vi "一致性测试确认.vi"(0 "Image In":T11=refnum, 1 "Image Dst":T11, 2 "ROI Descriptor (Find Straight Edge 1)":T4={"Global Rectangle"=[508, 1161, 875, 1411], "Contours"=[{"ID"=enum."External", "Type"=12, "Coordinates"=[508, 1161, 875, 1411, 0]}]} {"Contours"."Type" items=["No Selection", "Point", "Line", "Rectangle", "Oval", "Polygon", "Freehand Region", "Annulus", "Unused2", "Unused3", "Broken Line", "Freehand Line", "Rotated Rectangle"]}, 3 "Options (Find Straight Edge 1)":T9={"Search Direction"=0, "Edge Options"={"Edge Polarity"=0, "Kernel Size"=9, "Width"=25, "Minimum Edge Strength"=47.0, "Interpolation Type"=enum."Bilinear Fixed", "Data Processing Method"=enum."Average"}, "Show Search Area"=TRUE, "Show Search Lines"=FALSE, "Show Edges Found"=FALSE, "Show Result"=TRUE, "Search Area Color"=6618880, "Search Lines Color"=16860, "Edge Locations Color"=6618880, "Result Color"=16711680, "Overlay Group Name"=""} {"Search Direction" items=["Left to Right", "Right to Left", "Top to Bottom", "Bottom to Top"]; "Edge Options"."Edge Polarity" items=["All Edges", "Rising Edges", "Falling Edges"]; "Edge Options"."Minimum Edge Strength" format="%.2f"; "Edge Options"."Width" step=2; "Edge Options"."Kernel Size" step=2}, 4 "Fit Options (Find Straight Edge 1)":T5={"Number of Lines"=1, "Type"=enum."First Edge Rake", "Min. Score"=10.0, "Max. Score"=1000.0, "Orientation"=0.0, "Angle Range"=45.0, "Angle Tolerance"=1.0, "Step Size"=12, "Min. SNR (db)"=0.0, "Min. Points (%)"=25.0, "Hough Iterations"=5} {"Min. Points (%)" min=0.0 max=100.0; "Min. SNR (db)" min=0.0; "Max. Score" min=0.0 max=1024.0; "Min. Score" min=0.0 max=1024.0 step=1.0}, 5 "ROI Descriptor (Edge Detector 1)":T4={"Global Rectangle"=[710, 1241, 2012, 1251], "Contours"=[{"ID"=enum."External", "Type"=2, "Coordinates"=[710, 1250, 2011, 1241]}]} {"Contours"."Type" items=["No Selection", "Point", "Line", "Rectangle", "Oval", "Polygon", "Freehand Region", "Annulus", "Unused2", "Unused3", "Broken Line", "Freehand Line", "Rotated Rectangle"]}, 6 "Process (Edge Detector 1)":T3(ring)=enum."Get All Edges", 7 "error in":errorcluster, 8 "Edge Options (Edge Detector 1)":T2={"Edge Polarity"=0, "Kernel Size"=9, "Width"=25, "Minimum Edge Strength"=47.0, "Interpolation Type"=enum."Bilinear Fixed", "Data Processing Method"=enum."Average"} {"Edge Polarity" items=["All Edges", "Rising Edges", "Falling Edges"]}, 9 "Algorithm (Pattern Matching 1)":i32(ring)=2 items=["All", "Low Discrepancy Sampling", "Grayscale Value Pyramid", "Gradients Pyramid"], 10 "Parameters (Pattern Matching 1)":T10={"Number of Matches Requested"=1, "Minimum Match Score"=699.0, "Angle Ranges"=[{"Start Angle"=-20.0, "End Angle"=20.0}]}, 11 "Template File Path (Pattern Matching 1)":path=path "D:/Inspect System/Source Code/Template Program/一致性模板.png", 12 "ROI Descriptor (Find Straight Edge 2)":T4={"Global Rectangle"=[1843, 1112, 2152, 1339], "Contours"=[{"ID"=enum."External", "Type"=12, "Coordinates"=[1844, 1113, 2151, 1338, -262]}]} {"Contours"."Type" items=["No Selection", "Point", "Line", "Rectangle", "Oval", "Polygon", "Freehand Region", "Annulus", "Unused2", "Unused3", "Broken Line", "Freehand Line", "Rotated Rectangle"]}, 13 "Options (Find Straight Edge 2)":T9={"Search Direction"=1, "Edge Options"={"Edge Polarity"=1, "Kernel Size"=7, "Width"=1, "Minimum Edge Strength"=51.0, "Interpolation Type"=enum."Bilinear Fixed", "Data Processing Method"=enum."Average"}, "Show Search Area"=TRUE, "Show Search Lines"=FALSE, "Show Edges Found"=FALSE, "Show Result"=TRUE, "Search Area Color"=65280, "Search Lines Color"=255, "Edge Locations Color"=16776960, "Result Color"=16711680, "Overlay Group Name"=""} {"Search Direction" items=["Left to Right", "Right to Left", "Top to Bottom", "Bottom to Top"]; "Edge Options"."Edge Polarity" items=["All Edges", "Rising Edges", "Falling Edges"]; "Edge Options"."Minimum Edge Strength" format="%.2f"; "Edge Options"."Width" step=2; "Edge Options"."Kernel Size" step=2}, 14 "Fit Options (Find Straight Edge 2)":T5={"Number of Lines"=1, "Type"=enum."First Edge Rake", "Min. Score"=10.0, "Max. Score"=1000.0, "Orientation"=0.0, "Angle Range"=45.0, "Angle Tolerance"=1.0, "Step Size"=7, "Min. SNR (db)"=0.0, "Min. Points (%)"=25.0, "Hough Iterations"=5} {"Min. Points (%)" min=0.0 max=100.0; "Min. SNR (db)" min=0.0; "Max. Score" min=0.0 max=1024.0; "Min. Score" min=0.0 max=1024.0 step=1.0}) -> (20 "Image Out":T11, 21 "Edge Information (Edge Detector 1)":T12[](array[typedef])=[{"Location (Pixel)"={"X"=1992.7675, "Y"=1249.6696}, "Location (Real-World)"={"X"=1992.7675, "Y"=1249.6696}, "Distance (Pixel)"=1243.7788960188627, "Distance (Real-World)"=1243.7788960188627, "Strength"=48.61714285714286, "Noise"=33.48, "Rising?"=FALSE}, {"Location (Pixel)"={"X"=2093.2168, "Y"=1249.239}, "Location (Real-World)"={"X"=2093.2168, "Y"=1249.239}, "Distance (Pixel)"=1344.2292914241552, "Distance (Real-World)"=1344.2292914241552, "Strength"=135.82857142857142, "Noise"=25.725714285714286, "Rising?"=FALSE}] {"Distance (Real-World)" format="%.2f"; "Location (Real-World)"."Y" format="%.2g"; "Location (Real-World)"."X" format="%.2f"; "Noise" format="%.2f"; "Location (Pixel)"."Y" format="%.2g"; "Location (Pixel)"."X" format="%.2f"; "Strength" format="%.2f"; "Distance (Pixel)" format="%.2f"}, 22 "Straight Edge (Find Straight Edge 1)":T13={"Point1 (Pixels)"={"X"=694.03955, "Y"=1165.1874}, "Point2 (Pixels)"={"X"=693.5, "Y"=1405.0}, "Point1 (Real-World)"={"X"=694.03955, "Y"=1165.1874}, "Point2 (Real-World)"={"X"=693.5, "Y"=1405.0}, "Angle (Pixel)"=-0.12890037757524908, "Angle (Real-World)"=-0.12890037757524908, "Score"=261.62465413411456, "Straightness"=0.11302218027687676, "Average SNR (db)"=31.042020668112016, "Calibration Valid"=TRUE} {"Point2 (Real-World)"."Y" format="%.2f"; "Point2 (Real-World)"."X" format="%.2f"; "Point1 (Real-World)"."Y" format="%.2f"; "Point1 (Real-World)"."X" format="%.2f"; "Point2 (Pixels)"."Y" format="%.2f"; "Point2 (Pixels)"."X" format="%.2f"; "Point1 (Pixels)"."Y" format="%.2f"; "Point1 (Pixels)"."X" format="%.2f"}, 23 "Matches (Pattern Matching 1)":T14(array[cluster])=[{"Position"={"x"=1379.1647, "y"=1245.8256}, "Angle"=0.08344074, "Scale"=1.0, "Score"=860.556, "Bounding Box"=[{"x"=653.5562, "y"=1171.8822}, {"x"=2104.5547, "y"=1169.7692}, {"x"=2104.773, "y"=1319.7689}, {"x"=653.7747, "y"=1321.882}, {"x"=653.5562, "y"=1171.8822}]}] {"Bounding Box"."y" format="%.2f"; "Bounding Box"."x" format="%.2f"; "Position"."y" format="%.2f"; "Position"."x" format="%.2f"; "Score" format="%.2f"; "Scale" format="%.2f"; "Angle" format="%.2f"}, 24 "Straight Edge (Find Straight Edge 2)":T13={"Point1 (Pixels)"={"X"=2089.7798, "Y"=1115.0}, "Point2 (Pixels)"={"X"=2095.6719, "Y"=1339.0}, "Point1 (Real-World)"={"X"=2089.7798, "Y"=1115.0}, "Point2 (Real-World)"={"X"=2095.6719, "Y"=1339.0}, "Angle (Pixel)"=1.5067815290214939, "Angle (Real-World)"=1.5067815290214939, "Score"=227.45098039215685, "Straightness"=2.5179862328858427, "Average SNR (db)"=23.738052089260176, "Calibration Valid"=TRUE} {"Point2 (Real-World)"."Y" format="%.2f"; "Point2 (Real-World)"."X" format="%.2f"; "Point1 (Real-World)"."Y" format="%.2f"; "Point1 (Real-World)"."X" format="%.2f"; "Point2 (Pixels)"."Y" format="%.2f"; "Point2 (Pixels)"."X" format="%.2f"; "Point1 (Pixels)"."Y" format="%.2f"; "Point1 (Pixels)"."X" format="%.2f"}, 25 "输出簇":T1={"Start X"=694, "Start Y"=1250, "End X"=2093, "End Y"=1241} {"Start X" scale=0.0..1024.0; "End X" scale=0.0..1024.0}, 27 "error out":errorcluster)   [LabVIEW 2017]
doc: "Creates, edits, and runs vision algorithms using NI Vision Assistant.\n\nWhen you place this Express VI on the block diagram, NI Vision Assistant launches. Create an algorithm using the Vision Assistant processing functions. After you create an algorithm, you can select the controls and indicators that you want to be able to programmatically set in LabVIEW. Double-click the Vision Assistant Express VI to edit the algorithm."
uses:
  <vilib>/vision/Image Controls.llb/IMAQ Image.ctl
  <vilib>/vision/Measure.llb/Edge New.ctl
  <vilib>/vision/Measure.llb/Edge Options.ctl
  <vilib>/vision/Measure.llb/Edge Polarity.ctl
  <vilib>/vision/Measure.llb/Straight Edge Options.ctl
  <vilib>/vision/Measure.llb/Straight Edge Process.ctl
  <vilib>/vision/NI_Vision_Development_Module.lvlib
panel:
  out "end X":sgl=2092.7258
  out "start X":sgl=693.7698
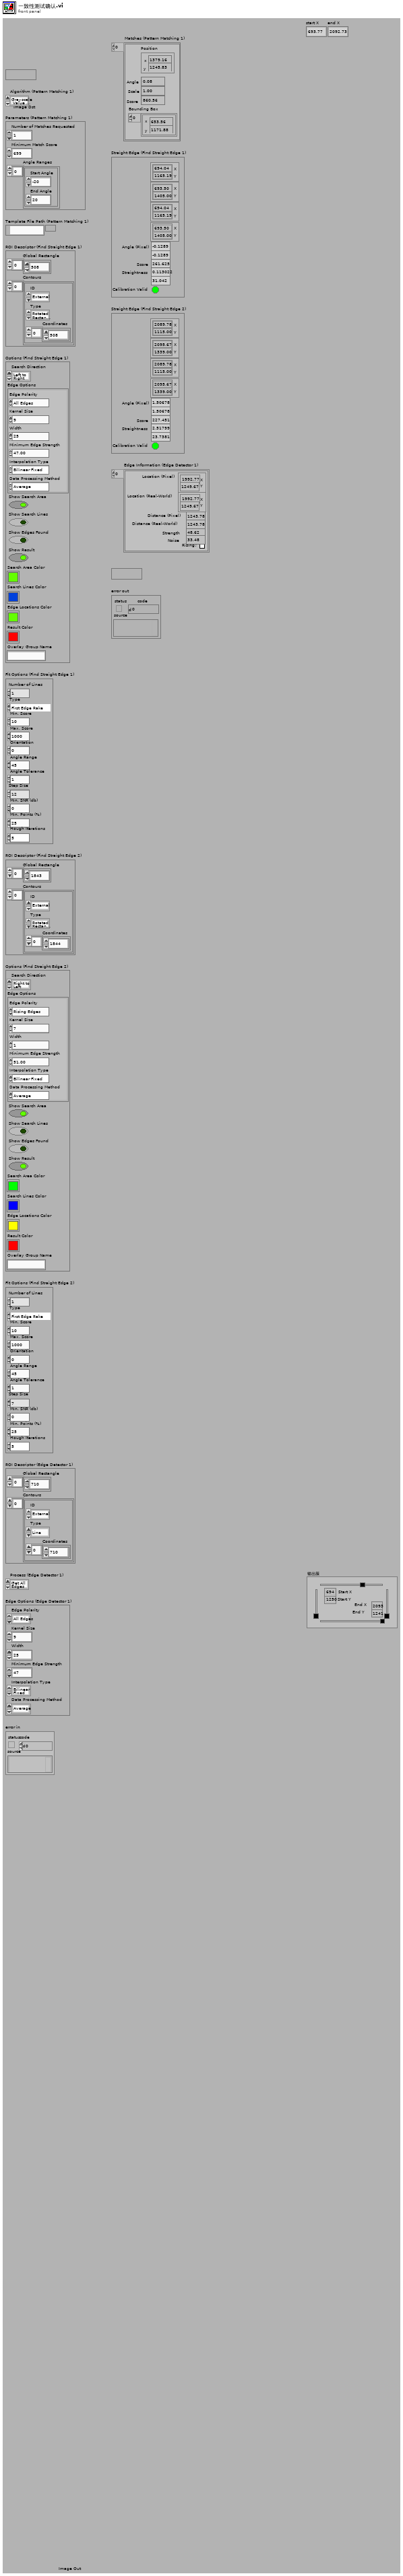
[diagram p1: front panel]
types:
  T1 = typedef "IMAQ Line" = cluster{"Start X":i32, "Start Y":i32, "End X":i32, "End Y":i32}
  T2 = cluster{"Edge Polarity":u32, "Kernel Size":u32, "Width":u32, "Minimum Edge Strength":sgl, "Interpolation Type":enum32{"Zero Order", "Bilinear", "Quadratic", "Cubic", "Bilinear Fixed"}, "Data Processing Method":enum32{"Average", "Median"}}
  T3 = enum16{"Get First Edge", "Get First + Last Edge", "Get All Edges", "Get Best Edge"}
  T4 = cluster{"Global Rectangle":i32[], "Contours":cluster{"ID":enum32{"External", "Internal"}, "Type":u32, "Coordinates":i32[]}[]}
  T5 = typedef "Straight Edge Options.ctl" = cluster{"Number of Lines":i32, "Type":T6, "Min. Score":dbl, "Max. Score":dbl, "Orientation":dbl, "Angle Range":dbl, "Angle Tolerance":dbl, "Step Size":u32, "Min. SNR (db)":dbl, "Min. Points (%)":dbl, "Hough Iterations":i32}
  T6 = typedef "Straight Edge Process.ctl" = enum32{"First Edge Rake", "Best Edge Rake", "Hough Edge Rake", "First Edge Projection", "Best Edge Projection"}
  T7 = typedef "Edge Options.ctl" = cluster{"Edge Polarity":T8, "Kernel Size":u32, "Width":u32, "Minimum Edge Strength":sgl, "Interpolation Type":enum32{"Zero Order", "Bilinear", "Quadratic", "Cubic", "Bilinear Fixed"}, "Data Processing Method":enum32{"Average", "Median"}}
  T8 = typedef "Edge Polarity.ctl" = u32
  T9 = cluster{"Search Direction":u32, "Edge Options":T7, "Show Search Area":bool, "Show Search Lines":bool, "Show Edges Found":bool, "Show Result":bool, "Search Area Color":u32, "Search Lines Color":u32, "Edge Locations Color":u32, "Result Color":u32, "Overlay Group Name":string}
  T10 = cluster{"Number of Matches Requested":i32, "Minimum Match Score":sgl, "Angle Ranges":cluster{"Start Angle":sgl, "End Angle":sgl}[]}
  T11 = typedef "IMAQ Image.ctl" = refnum<image>
  T12 = typedef "Edge New.ctl" = cluster{"Location (Pixel)":cluster{"X":sgl, "Y":sgl}, "Location (Real-World)":cluster{"X":sgl, "Y":sgl}, "Distance (Pixel)":dbl, "Distance (Real-World)":dbl, "Strength":dbl, "Noise":dbl, "Rising?":bool}
  T13 = cluster{"Point1 (Pixels)":cluster{"X":sgl, "Y":sgl}, "Point2 (Pixels)":cluster{"X":sgl, "Y":sgl}, "Point1 (Real-World)":cluster{"X":sgl, "Y":sgl}, "Point2 (Real-World)":cluster{"X":sgl, "Y":sgl}, "Angle (Pixel)":dbl, "Angle (Real-World)":dbl, "Score":dbl, "Straightness":dbl, "Average SNR (db)":dbl, "Calibration Valid":bool}
  T14 = cluster{"Position":cluster{"x":sgl, "y":sgl}, "Angle":sgl, "Scale":sgl, "Score":sgl, "Bounding Box":cluster{"x":sgl, "y":sgl}[]}[]
  T15 = cluster{"Origin":cluster{"X":sgl, "Y":sgl}, "Angle (deg)":sgl, "Axis Reference":u32}
  T16 = enum16{"Reset", "Update Coordinate System", "Get Coordinate System"}
  T17 = enum16{"Horizontal Motion", "Vertical Motion", "Horizontal and Vertical Motion", "Horizontal, Vertical and Angular Motion"}
  T18 = typedef "Image Type" = u32
  T19 = typedef "IMAQ Coordinate System" = cluster{"Reference System":cluster{"Origin":cluster{"X":sgl, "Y":sgl}, "Angle (deg)":sgl, "Axis Reference":u32}, "Measurement System":cluster{"Origin":cluster{"X":sgl, "Y":sgl}, "Angle (deg)":sgl, "Axis Reference":u32}}
  T20 = typedef "ROI Descriptor" = cluster{"Global Rectangle":i32[], "Contours":cluster{"ID":enum32{"External", "Internal"}, "Type":u32, "Coordinates":i32[]}[]}
  T21 = cluster{"Point1 (Pixels)":cluster{"X":sgl, "Y":sgl}, "Point2 (Pixels)":cluster{"X":sgl, "Y":sgl}, "Point1 (Real-World)":cluster{"X":sgl, "Y":sgl}, "Point2 (Real-World)":cluster{"X":sgl, "Y":sgl}, "Angle (Pixel)":dbl, "Angle (Real-World)":dbl, "Score":dbl, "Straightness":dbl, "Average SNR (db)":dbl, "Calibration Valid":bool}[]
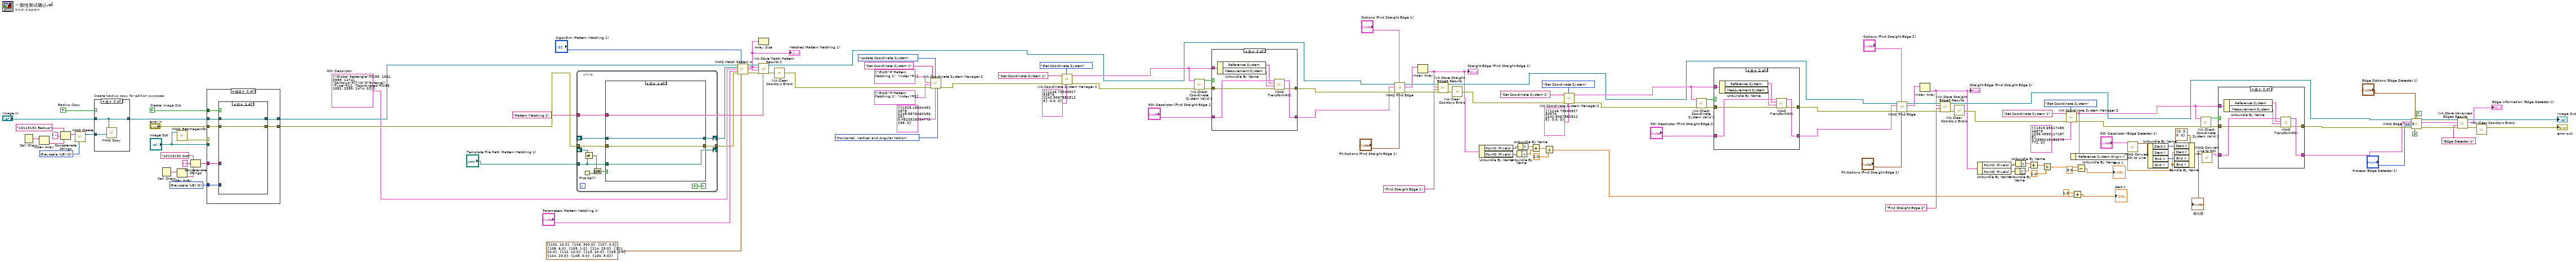
[diagram p0: block diagram]
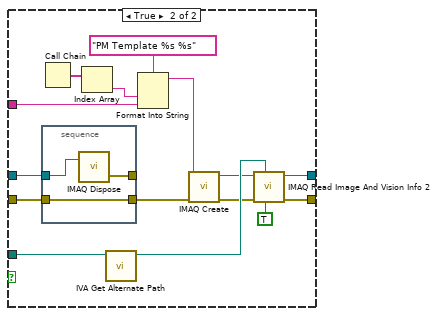
[diagram p5: hidden frame]
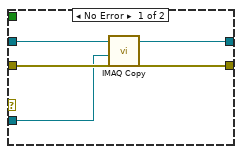
[diagram p6: hidden frame]
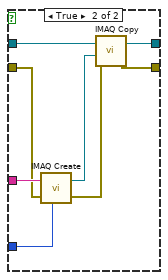
[diagram p7: hidden frame]
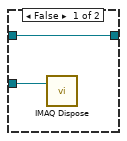
[diagram p8: hidden frame]
diagram:
  w103 = "Pattern Matching 1" ("Step Name")
  w105 = T4 {"Global Rectangle"=[295, 1061, 2595, 1474], "Contours"=[{"ID"=enum."External", "Type"=12, "Coordinates"=[295, 1061, 2595, 1474, 0]}]}  # ROI Descriptor
  w111 = T18 0 items=["Grayscale (U8)", "Grayscale (I16)", "Grayscale (SGL)", "Complex (CSG)", "RGB (U32)", "HSL (U32)", "RGB (U64)", "Grayscale (U16)"] ("Image Dst Type")
  w112 = T18 0 items=["Grayscale (U8)", "Grayscale (I16)", "Grayscale (SGL)", "Complex (CSG)", "RGB (U32)", "HSL (U32)", "RGB (U64)", "Grayscale (U16)"] ("Image Type")
  w131 = TRUE  # Backup Copy
  w124 = FALSE  # Create Image Dst
  n1 = Call Chain() -> (call chain=w118:string[])
  n2 = Index Array(array=w118) -> (element=w117:string)  [unwired: 1 in]
  n3 = Concatenate Strings("10113132 Backup" ("Backup Image Name"), " ", w117) -> (w114:string)
  n4 = call "IMAQ Create"("Image Name"=w114, "Image Type"=w112) -> ("New Image"=w113:T11)  [unwired: 2 in, 2 out]
  n5 = case "Create backup copy for edition purposes" shown="真" w131 {
    tunnel: [w133 w135] -> w127
    tunnel: "Image In" -> [w133 w135]
    tunnel: w113 -> [w132 w134]
    frame False {
      n6 = call "IMAQ Dispose"("Image"=w132) -> ()  [unwired: 2 in, 4 out]
    }
    frame True {
      n7 = call "IMAQ Copy"("Image Dst"=w134, "Image Src"=w135) -> ()  [unwired: 1 in, 5 out]
    }
  }
  n8 = Call Chain() -> (call chain=w123:string[])
  n9 = call "IMAQ GetImageInfo"("Image"="Image Dst") -> ("error out"=w129:errorcluster)  [unwired: 1 in, 9 out]
  n10 = Index Array(array=w123) -> (element=w121:string)  [unwired: 1 in]
  n11 = Concatenate Strings("10113132 Dst" ("Image Dst Name"), " ", w121) -> (w119:string)
  n12 = case "条件结构" shown="错误" w129 {
    tunnel: [w140 w144] -> w109
    tunnel: [w139 w143] -> w125
    tunnel: w127 -> [w138 w145]
    tunnel: "error in" -> [w137 w141]
    tunnel: "Image Dst" -> [w136 _]
    tunnel: w119 -> [_ w147]
    tunnel: w111 -> [_ w146]
    tunnel: w124 -> [_ w142]
    frame No Error {
      n13 = call "IMAQ Copy"("error in (no error)"=w137, "Image Dst"=w136, "Image Src"=w138) -> ("error out"=w139:errorcluster, "Image Dst Out"=w140:T11)  [unwired: 3 out]
    }
    frame Error {
      n14 = case "条件结构" shown="假" w142 {
        tunnel: w147 -> [_ w157]
        tunnel: w146 -> [_ w156]
        tunnel: w145 -> [w149 w154]
        tunnel: [w149 w153] -> w144
        tunnel: [w148 w152] -> w143
        tunnel: w141 -> [w148 w150]
        frame False {
        }
        frame True {
          n15 = call "IMAQ Create"("Image Name"=w157, "Image Type"=w156, "error in (no error)"=w150) -> ("New Image"=w155:T11, "error out"=w151:errorcluster)  [unwired: 1 in, 1 out]
          n16 = call "IMAQ Copy"("error in (no error)"=w151, "Image Dst"=w155, "Image Src"=w154) -> ("error out"=w152:errorcluster, "Image Dst Out"=w153:T11)  [unwired: 3 out]
        }
      }
    }
  }
  n17 = while {
    shift-right: [w168] -> w100
    shift-left: _ -> [w167]
    tunnel: [w165] -> w99
    tunnel: w125 -> [w164]
    tunnel: "Template File Path (Pattern Matching 1)" -> [w161]
    tunnel: w103 -> [w163]
    shift-right: [w161] -> _
    shift-left: _ -> [w162]
    stop <- FALSE continue-if-true
    n18 = First Call?() -> (First Call?: T/F=w160:bool)
    n19 = Not Equal?(x=w162, y=w161) -> (x != y?=w159:bool)
    n20 = Or(x=w159, y=w160) -> (x .or. y?=w158:bool)
    n21 = case "条件结构" shown="假" w158 {
      tunnel: [w170 w175] -> w168
      tunnel: w167 -> [w170 w179]
      tunnel: [w169 w176] -> w165
      tunnel: w164 -> [w169 w178]
      tunnel: w161 -> [_ w180]
      tunnel: w163 -> [_ w181]
      frame False {
      }
      frame True {
        n22 = stacked-sequence "层叠式顺序结构" {
          tunnel: w179 -> [w188]
          tunnel: w178 -> [w187]
          tunnel: [w187] -> w172
          tunnel: [w186] -> _
          frame #0 {
            n23 = call "IMAQ Dispose"("Image"=w188) -> ("error out"=w186:errorcluster)  [unwired: 2 in, 3 out]
          }
        }
        n24 = Call Chain() -> (call chain=w183:string[])
        n25 = Index Array(array=w183) -> (element=w182:string)  [unwired: 1 in]
        n26 = call <vilib>:"IVA Get Alternate Path.vi"("Path In"=w180) -> ("Path Out"=w177:path)  [unwired: 10 out]
        n27 = Format Into String(format string="PM Template %s %s" ("Image Name"), w182, w181) -> (resulting string=w185:string)  [unwired: 2 in, 1 out]
        n28 = call "IMAQ Create"("Image Name"=w185, "error in (no error)"=w172) -> ("New Image"=w174:T11, "error out"=w173:errorcluster)  [unwired: 2 in, 1 out]
        n29 = call "IMAQ Read Image And Vision Info 2"("Use File Path Image Type"=TRUE, "File Path"=w177, "error in (no error)"=w173, "Image"=w174) -> ("error out"=w176:errorcluster, "Image Out"=w175:T11)  [unwired: 5 in, 1 out]
      }
    }
  }
  n30 = call "IMAQ Match Pattern 4"("Image"=w109, "Algorithm"="Algorithm (Pattern Matching 1)", "Template Image"=w100, "ROI Descriptor"=w105, "Parameters"="Parameters (Pattern Matching 1)", "error in (no error)"=w99, "Advanced Options"=cluster{"Item":u16, "Value":dbl}[] [{"Item"=102, "Value"=10.0}, {"Item"=106, "Value"=300.0}, {"Item"=107, "Value"=0.0}, {"Item"=108, "Value"=6.0}, {"Item"=109, "Value"=1.0}, {"Item"=114, "Value"=25.0}, {"Item"=111, "Value"=20.0}, {"Item"=112, "Value"=10.0}, {"Item"=113, "Value"=20.0}, {"Item"=103, "Value"=1.0}, {"Item"=104, "Value"=20.0}, {"Item"=105, "Value"=0.0}, {"Item"=100, "Value"=5.0}]) -> ("Image (duplicate)"=w107:T11, "Matches (pixel)"=w102:T14, "Matches (real-world)"=w101:T14, "error out"=w108:errorcluster)  [unwired: 4 in, 1 out]
  "Matches (Pattern Matching 1)" <- w102
  n31 = Array Size(array=w102) -> ()  [unwired: 1 out]
  n32 = call <vilib>:"IVA Store Match Pattern Results 2.vi"("Step Name"=w103, "error in (no error)"=w108, "Matches (real-world)"=w101, "Matches (pixel)"=w102, "Image in"=w107) -> ("error out"=w98:errorcluster, "Image dup"=w79:T11)  [unwired: 1 in, 4 out]
  n33 = call <vilib>:"IVA Clear Coordsys Errors.vi"("error in (no error)"=w98) -> ("error out"=w97:errorcluster)  [unwired: 10 in]
  n34 = call <vilib>:"IVA Coordinate System Manager 2.vi"("Mode"=T17."Horizontal, Vertical and Angular Motion", "Reference System"=T15 {"Origin"={"X"=1329.196, "Y"=1248.8577}, "Angle (deg)"=0.45203266, "Axis Reference"=0}, "Function"=T16."Update Coordinate System", "error in (no error)"=w97, "Angle ID"=cluster{"GUID":string, "Index":i32} {"GUID"="Pattern Matching 1", "Index"=3}, "Origin ID"=cluster{"GUID":string, "Index":i32} {"GUID"="Pattern Matching 1", "Index"=1}, "Coordinate System Name"="Set Coordinate System 1") -> ("error out"=w89:errorcluster)  [unwired: 4 out]
  n35 = call <vilib>:"IVA Coordinate System Manager 2.vi"("Reference System"=T15 {"Origin"={"X"=1246.7904, "Y"=1242.9067}, "Angle (deg)"=0.0, "Axis Reference"=0}, "Function"=T16."Get Coordinate System", "error in (no error)"=w89, "Coordinate System Name"="Set Coordinate System 1") -> ("error out"=w86:errorcluster, "Coordinate System Out"=w82:T19)  [unwired: 3 in, 3 out]
  n36 = call <vilib>:"IVA Check Coordinate System Valid 2.vi"("error in (no error)"=w86, "Coordinate System"=w82) -> ("error out"=w80:errorcluster, "Valid?"=w81:bool)  [unwired: 8 out]
  n37 = case "条件结构" shown="真" w81 {
    tunnel: "ROI Descriptor (Find Straight Edge 1)" -> [w190 w197]
    tunnel: [w190 w194] -> w78
    tunnel: [w189 w193] -> w83
    tunnel: w82 -> [_ w192]
    tunnel: w80 -> [w189 w191]
    frame False {
    }
    frame True {
      n38 = Unbundle By Name(w192) -> ("Reference System"=w196:T15, "Measurement System"=w195:T15)
      n39 = call "IMAQ TransformROI"("error in (no error)"=w191, "New Reference"=w195, "Base Reference"=w196, "ROI Descriptor"=w197) -> ("error out"=w193:errorcluster, "ROI Descriptor out"=w194:T20)  [unwired: 6 out]
    }
  }
  n40 = call "IMAQ Find Edge"("Line Fit Options"="Fit Options (Find Straight Edge 1)", "Options"="Options (Find Straight Edge 1)", "error in (no error)"=w83, "ROI Descriptor"=w78, "Image"=w79) -> ("error out"=w73:errorcluster, "Straight Edges"=w72:T21, "Image Out"=w74:T11)  [unwired: 1 in, 3 out]
  n41 = Index Array(array=w72) -> (element=w24:T13)  [unwired: 1 in]
  "Straight Edge (Find Straight Edge 1)" <- w24
  n42 = call <vilib>:"IVA Store Straight Edge3 Results.vi"("error in (no error)"=w73, "Step Name"="Find Straight Edge 1", "Straight Edge"=w24, "Image in"=w74) -> ("error out"=w71:errorcluster, "Image dup"=w60:T11)  [unwired: 1 in, 5 out]
  n43 = call <vilib>:"IVA Clear Coordsys Errors.vi"("error in (no error)"=w71) -> ("error out"=w70:errorcluster)  [unwired: 10 in]
  n44 = Unbundle By Name(w24) -> ("Point1 (Pixels)"=w29:cluster{"X":sgl, "Y":sgl}, "Point2 (Pixels)"=w28:cluster{"X":sgl, "Y":sgl})
  n45 = Unbundle By Name(w28) -> ("X"=w26:sgl)
  n46 = Unbundle By Name(w29) -> ("X"=w27:sgl)
  n47 = Add(x=w27, y=w26) -> (x+y=w25:sgl)
  n48 = Divide(x=w25, y=sgl 2.0) -> (x/y=w10:sgl)
  n49 = call <vilib>:"IVA Coordinate System Manager 2.vi"("Reference System"=T15 {"Origin"={"X"=1246.7904, "Y"=1242.9067}, "Angle (deg)"=0.0, "Axis Reference"=0}, "Function"=T16."Get Coordinate System", "error in (no error)"=w70, "Coordinate System Name"="Set Coordinate System 1") -> ("error out"=w67:errorcluster, "Coordinate System Out"=w63:T19)  [unwired: 3 in, 3 out]
  n50 = call <vilib>:"IVA Check Coordinate System Valid 2.vi"("error in (no error)"=w67, "Coordinate System"=w63) -> ("error out"=w61:errorcluster, "Valid?"=w62:bool)  [unwired: 8 out]
  n51 = case "条件结构" shown="真" w62 {
    tunnel: "ROI Descriptor (Find Straight Edge 2)" -> [w199 w206]
    tunnel: [w199 w203] -> w59
    tunnel: [w198 w202] -> w64
    tunnel: w63 -> [_ w201]
    tunnel: w61 -> [w198 w200]
    frame False {
    }
    frame True {
      n52 = Unbundle By Name(w201) -> ("Reference System"=w205:T15, "Measurement System"=w204:T15)
      n53 = call "IMAQ TransformROI"("error in (no error)"=w200, "New Reference"=w204, "Base Reference"=w205, "ROI Descriptor"=w206) -> ("error out"=w202:errorcluster, "ROI Descriptor out"=w203:T20)  [unwired: 6 out]
    }
  }
  n54 = call "IMAQ Find Edge"("Line Fit Options"="Fit Options (Find Straight Edge 2)", "Options"="Options (Find Straight Edge 2)", "error in (no error)"=w64, "ROI Descriptor"=w59, "Image"=w60) -> ("error out"=w54:errorcluster, "Straight Edges"=w53:T21, "Image Out"=w55:T11)  [unwired: 1 in, 3 out]
  n55 = Index Array(array=w53) -> (element=w16:T13)  [unwired: 1 in]
  "Straight Edge (Find Straight Edge 2)" <- w16
  n56 = call <vilib>:"IVA Store Straight Edge3 Results.vi"("error in (no error)"=w54, "Step Name"="Find Straight Edge 2", "Straight Edge"=w16, "Image in"=w55) -> ("error out"=w52:errorcluster, "Image dup"=w43:T11)  [unwired: 1 in, 5 out]
  n57 = call <vilib>:"IVA Clear Coordsys Errors.vi"("error in (no error)"=w52) -> ("error out"=w51:errorcluster)  [unwired: 10 in]
  n58 = Unbundle By Name(w16) -> ("Point1 (Pixels)"=w17:cluster{"X":sgl, "Y":sgl}, "Point2 (Pixels)"=w18:cluster{"X":sgl, "Y":sgl})
  n59 = Unbundle By Name(w18) -> ("X"=w20:sgl)
  n60 = Unbundle By Name(w17) -> ("X"=w19:sgl)
  n61 = Add(x=w19, y=w20) -> (x+y=w21:sgl)
  n62 = Divide(x=w21, y=sgl 2.0) -> (x/y=w11:sgl)
  n63 = call <vilib>:"IVA Coordinate System Manager 2.vi"("Reference System"=T15 {"Origin"={"X"=1323.6542, "Y"=1239.4995}, "Angle (deg)"=0.23892452, "Axis Reference"=0}, "Function"=T16."Get Coordinate System", "error in (no error)"=w51, "Coordinate System Name"="Set Coordinate System 1") -> ("error out"=w48:errorcluster, "Coordinate System Out"=w4:T19)  [unwired: 3 in, 3 out]
  n64 = Unbundle By Name(w4) -> ("Reference System.Origin.Y"=w3:sgl)
  n65 = Add(x=sgl 1.0, y=w10) -> (x+y=→"start X":sgl)
  n66 = Subtract(x=w11, y=sgl 5.0) -> (x-y=→"end X":sgl)
  n67 = call "IMAQ Convert ROI to Line"("ROI Descriptor"="ROI Descriptor (Edge Detector 1)") -> ("Line"=w14:T1)  [unwired: 8 in, 1 out]
  n68 = Unbundle By Name(w14) -> ("Start X"=w2:i32, "End X"=w1:i32)  [unwired: 2 out]
  n69 = Bundle By Name(cluster=T1 {"Start X"=0, "Start Y"=0, "End X"=0, "End Y"=0} ("Line"), "Start X"=w2, "Start Y"=w3, "End X"=w1, "End Y"=w3) -> (w13:T1)
  "输出簇" <- w13
  n70 = call <vilib>:"IVA Check Coordinate System Valid 2.vi"("error in (no error)"=w48, "Coordinate System"=w4) -> ("error out"=w44:errorcluster, "Valid?"=w45:bool)  [unwired: 8 out]
  n71 = call "IMAQ Convert Line to ROI"("Line"=w13) -> ("ROI Descriptor"=w9:T20)  [unwired: 8 in, 1 out]
  n72 = case "条件结构" shown="真" w45 {
    tunnel: w9 -> [w208 w215]
    tunnel: [w208 w212] -> w35
    tunnel: [w207 w211] -> w46
    tunnel: w4 -> [_ w210]
    tunnel: w44 -> [w207 w209]
    frame False {
    }
    frame True {
      n73 = Unbundle By Name(w210) -> ("Reference System"=w214:T15, "Measurement System"=w213:T15)
      n74 = call "IMAQ TransformROI"("error in (no error)"=w209, "New Reference"=w213, "Base Reference"=w214, "ROI Descriptor"=w215) -> ("error out"=w211:errorcluster, "ROI Descriptor out"=w212:T20)  [unwired: 6 out]
    }
  }
  n75 = call "IMAQ Edge Tool 3"("Image"=w43, "Edge Options"="Edge Options (Edge Detector 1)", "Optimized Mode"=TRUE, "ROI Descriptor"=w35, "Process"="Process (Edge Detector 1)", "error in (no error)"=w46, "Reverse Direction"=FALSE) -> ("Image (duplicate)"=w39:T11, "Edge Information"=w38:T12[], "error out"=w40:errorcluster)  [unwired: 6 out]
  n76 = call <vilib>:"IVA Store Advanced Edges Results.vi"("error in (no error)"=w40, "Step Name"="Edge Detector 1", "Edge Information"=w38, "Image in"=w39) -> ("error out"=w32:errorcluster, "Edge Information dup"=→"Edge Information (Edge Detector 1)":T12[], "Image dup"=→"Image Out":T11)  [unwired: 5 out]
  n77 = call <vilib>:"IVA Clear Coordsys Errors.vi"("error in (no error)"=w32) -> ("error out"=→"error out":errorcluster)  [unwired: 10 in]
